vi "HFRR ADV v042.vi"() -> ()   [LabVIEW 2025] (continued)
        n1342 = case shown="True" w1655 {
          selector: w1655 -> [_ w1662]
          frame False {
          }
          frame True {
            n1343 = Not(x=w1662) -> (.not. x?=w1661:bool)
            n1344 = local write "LIVE FEED MIN TEMP"(w1661) -> ()
            n1345 = call "CAMERA LIVE FEED FGV.vi"("Enum - Menu"=CAMERA_LIVE_FEED_ENUM."CAMERA MINIMIZE") -> ()  [unwired: 9 in, 2 out]
          }
        }
        n1346 = case shown="True" w1653 {
          selector: w1653 -> [_ w1659]
          frame False {
          }
          frame True {
            n1347 = Not(x=w1659) -> (.not. x?=w1658:bool)
            n1348 = local write "CAMERA ROI MIN TEMP"(w1658) -> ()
            n1349 = call "IMAGE ANALYSIS.vi"("Enum"=POST_ANALYSIS_ENUM."MINIMIZE UI") -> ()  [unwired: 9 in, 2 out]
          }
        }
        n1350 = local write "CAMERA ROI MAX TEMP"(TRUE ("CAMERA ROI MAX TEMP")) -> ()
      }
      frame "Adv Scar" {
        n1351 = local read "CAMERA ROI MIN TEMP"() -> (w1663:bool)
        n1352 = case shown="True" "LIVE FEED MAX TEMP" {
          selector: "LIVE FEED MAX TEMP" -> [_ w1684]
          frame False {
          }
          frame True {
            n1353 = Not(x=w1684) -> (.not. x?=w1683:bool)
            n1354 = local write "LIVE FEED MAX TEMP"(w1683) -> ()
            n1355 = call "CAMERA LIVE FEED FGV.vi"("Enum - Menu"=CAMERA_LIVE_FEED_ENUM."CAMERA RESTORE") -> ("error out"=w1674:errorcluster)  [unwired: 9 in, 1 out]
            n1356 = Type Cast(type=30, x=0) -> (*(type *) &x=w1678:i32)
            n1357 = Add(x=w1678, y=48) -> (x+y=w1679:i32)
            n1358 = call "CAMERA LIVE FEED FGV.vi"("Enum - Menu"=CAMERA_LIVE_FEED_ENUM."CAMERA MODE SET", "error in (no error)"=w1674, "CAMERA MODE"=w1679) -> ("error out"=w1671:errorcluster)  [unwired: 7 in, 1 out]
            n1359 = call "CAMERA LIVE FEED FGV.vi"("Enum - Menu"=CAMERA_LIVE_FEED_ENUM."CAMERA GRAY", "error in (no error)"=w1671) -> ("error out"=w1670:errorcluster)  [unwired: 8 in, 1 out]
            n1360 = call "LIST FILE NAMES.vi"("error in (no error)"=w1670) -> ("error out"=w1680:errorcluster, "filenames"=w1681:string[])  [unwired: 9 in]
            n1361 = property on="FILE 3" class="CmbBox"(error in=w1680, "Strings[]"=w1681) -> ()  [unwired: 1 in, 2 out]
          }
        }
        n1362 = case shown="True" w1663 {
          selector: w1663 -> [_ w1669]
          frame False {
          }
          frame True {
            n1363 = Not(x=w1669) -> (.not. x?=w1668:bool)
            n1364 = local write "CAMERA ROI MIN TEMP"(w1668) -> ()
            n1365 = call "IMAGE ANALYSIS.vi"("Enum"=POST_ANALYSIS_ENUM."MINIMIZE UI") -> ()  [unwired: 9 in, 2 out]
          }
        }
        n1366 = local write "CAMERA ROI MAX TEMP"(TRUE ("CAMERA ROI MAX TEMP")) -> ()
        "LIVE FEED MIN TEMP" <- TRUE ("LIVE FEED MIN TEMP")
      }
      frame "Adv Scar Report" {
        n1367 = local read "CAMERA ROI MAX TEMP"() -> (w1685:bool)
        n1368 = local read "LIVE FEED MIN TEMP"() -> (w1687:bool)
        n1369 = local write "LIVE FEED MAX TEMP"(TRUE ("LIVE FEED MAX TEMP")) -> ()
        n1370 = case shown="True" w1687 {
          selector: w1687 -> [_ w1696]
          frame False {
          }
          frame True {
            n1371 = Not(x=w1696) -> (.not. x?=w1695:bool)
            n1372 = local write "LIVE FEED MIN TEMP"(w1695) -> ()
            n1373 = call "CAMERA LIVE FEED FGV.vi"("Enum - Menu"=CAMERA_LIVE_FEED_ENUM."CAMERA MINIMIZE") -> ()  [unwired: 9 in, 2 out]
          }
        }
        n1374 = case shown="True" w1685 {
          selector: w1685 -> [_ w1693]
          frame False {
          }
          frame True {
            n1375 = Not(x=w1693) -> (.not. x?=w1691:bool)
            n1376 = local write "CAMERA ROI MAX TEMP"(w1691) -> ()
            n1377 = call "IMAGE ANALYSIS.vi"("Enum"=POST_ANALYSIS_ENUM."SHOW UI") -> ("error out"=w1690:errorcluster)  [unwired: 9 in, 1 out]
            n1378 = call "LIST FILE NAMES.vi"("error in (no error)"=w1690) -> ("filenames"=w1689:string[])  [unwired: 9 in, 1 out]
            n1379 = property on="Test File List :" class="CmbBox"("Strings[]"=w1689) -> ()  [unwired: 2 in, 2 out]
          }
        }
        n1380 = local write "CAMERA ROI MIN TEMP"(TRUE ("CAMERA ROI MIN TEMP")) -> ()
      }
      frame "Compare Files" {
        n1381 = local read "LIVE FEED MIN TEMP"() -> (w1699:bool)
        n1382 = local write "LIVE FEED MAX TEMP"(TRUE ("LIVE FEED MAX TEMP")) -> ()
        n1383 = local read "CAMERA ROI MIN TEMP"() -> (w1697:bool)
        n1384 = case shown="True" w1699 {
          selector: w1699 -> [_ w1706]
          frame False {
          }
          frame True {
            n1385 = Not(x=w1706) -> (.not. x?=w1705:bool)
            n1386 = local write "LIVE FEED MIN TEMP"(w1705) -> ()
            n1387 = call "CAMERA LIVE FEED FGV.vi"("Enum - Menu"=CAMERA_LIVE_FEED_ENUM."CAMERA MINIMIZE") -> ()  [unwired: 9 in, 2 out]
          }
        }
        n1388 = case shown="True" w1697 {
          selector: w1697 -> [_ w1703]
          frame False {
          }
          frame True {
            n1389 = Not(x=w1703) -> (.not. x?=w1702:bool)
            n1390 = local write "CAMERA ROI MIN TEMP"(w1702) -> ()
            n1391 = call "IMAGE ANALYSIS.vi"("Enum"=POST_ANALYSIS_ENUM."MINIMIZE UI") -> ()  [unwired: 9 in, 2 out]
          }
        }
        n1392 = local write "CAMERA ROI MAX TEMP"(TRUE ("CAMERA ROI MAX TEMP")) -> ()
      }
      frame "About" {
        n1393 = local read "LIVE FEED MIN TEMP"() -> (w1709:bool)
        n1394 = local write "LIVE FEED MAX TEMP"(TRUE ("LIVE FEED MAX TEMP")) -> ()
        n1395 = local read "CAMERA ROI MIN TEMP"() -> (w1708:bool)
        n1396 = case shown="True" w1709 {
          selector: w1709 -> [_ w1716]
          frame False {
          }
          frame True {
            n1397 = Not(x=w1716) -> (.not. x?=w1715:bool)
            n1398 = local write "LIVE FEED MIN TEMP"(w1715) -> ()
            n1399 = call "CAMERA LIVE FEED FGV.vi"("Enum - Menu"=CAMERA_LIVE_FEED_ENUM."CAMERA MINIMIZE") -> ()  [unwired: 9 in, 2 out]
          }
        }
        n1400 = case shown="True" w1708 {
          selector: w1708 -> [_ w1713]
          frame False {
          }
          frame True {
            n1401 = Not(x=w1713) -> (.not. x?=w1712:bool)
            n1402 = local write "CAMERA ROI MIN TEMP"(w1712) -> ()
            n1403 = call "IMAGE ANALYSIS.vi"("Enum"=POST_ANALYSIS_ENUM."MINIMIZE UI") -> ()  [unwired: 9 in, 2 out]
          }
        }
        n1404 = local write "CAMERA ROI MAX TEMP"(TRUE ("CAMERA ROI MIN TEMP")) -> ()
      }
      frame "Advance" {
        n1405 = local read "LIVE FEED MIN TEMP"() -> (w1719:bool)
        n1406 = local write "LIVE FEED MAX TEMP"(TRUE ("LIVE FEED MAX TEMP")) -> ()
        n1407 = local read "CAMERA ROI MIN TEMP"() -> (w1717:bool)
        n1408 = case shown="True" w1719 {
          selector: w1719 -> [_ w1726]
          frame False {
          }
          frame True {
            n1409 = Not(x=w1726) -> (.not. x?=w1725:bool)
            n1410 = local write "LIVE FEED MIN TEMP"(w1725) -> ()
            n1411 = call "CAMERA LIVE FEED FGV.vi"("Enum - Menu"=CAMERA_LIVE_FEED_ENUM."CAMERA MINIMIZE") -> ()  [unwired: 9 in, 2 out]
          }
        }
        n1412 = local write "CAMERA ROI MAX TEMP"(TRUE ("CAMERA ROI MAX TEMP")) -> ()
        n1413 = case shown="True" w1717 {
          selector: w1717 -> [_ w1723]
          frame False {
          }
          frame True {
            n1414 = Not(x=w1723) -> (.not. x?=w1722:bool)
            n1415 = local write "CAMERA ROI MIN TEMP"(w1722) -> ()
            n1416 = call "IMAGE ANALYSIS.vi"("Enum"=POST_ANALYSIS_ENUM."MINIMIZE UI") -> ()  [unwired: 9 in, 2 out]
          }
        }
      }
      frame "Mooha" {
        n1417 = local read "LIVE FEED MIN TEMP"() -> (w1729:bool)
        n1418 = local write "LIVE FEED MAX TEMP"(TRUE ("LIVE FEED MAX TEMP")) -> ()
        n1419 = local read "CAMERA ROI MIN TEMP"() -> (w1727:bool)
        n1420 = case shown="True" w1729 {
          selector: w1729 -> [_ w1736]
          frame False {
          }
          frame True {
            n1421 = Not(x=w1736) -> (.not. x?=w1735:bool)
            n1422 = local write "LIVE FEED MIN TEMP"(w1735) -> ()
            n1423 = call "CAMERA LIVE FEED FGV.vi"("Enum - Menu"=CAMERA_LIVE_FEED_ENUM."CAMERA MINIMIZE") -> ()  [unwired: 9 in, 2 out]
          }
        }
        n1424 = local write "CAMERA ROI MAX TEMP"(TRUE ("CAMERA ROI MAX TEMP")) -> ()
        n1425 = case shown="True" w1727 {
          selector: w1727 -> [_ w1733]
          frame False {
          }
          frame True {
            n1426 = Not(x=w1733) -> (.not. x?=w1732:bool)
            n1427 = local write "CAMERA ROI MIN TEMP"(w1732) -> ()
            n1428 = call "IMAGE ANALYSIS.vi"("Enum"=POST_ANALYSIS_ENUM."MINIMIZE UI") -> ()  [unwired: 9 in, 2 out]
          }
        }
      }
    }
    n1429 = local read "Auto Start Test"() -> (w1474:bool)
    n1430 = case shown="True" "sign in temp" {
      frame False {
      }
      frame True {
        w1509 = 1 ("y")
        n1431 = local read "USERNAME"() -> (w1515:string)
        n1432 = local read "USER ID"() -> (w1512:string)
        n1433 = call <vilib>:"Trim Whitespace.vi"("string"=w1515) -> ("trimmed string"=w1514:string)  [unwired: 1 in]
        n1434 = call <vilib>:"Trim Whitespace.vi"("string"=w1512) -> ("trimmed string"=w1513:string)  [unwired: 1 in]
        n1435 = String Length(string=w1514) -> (length=w1511:i32)
        n1436 = String Length(string=w1513) -> (length=w1510:i32)
        n1437 = Greater?(x=w1511, y=w1509) -> (0:w1508:bool)
        n1438 = Greater?(x=w1510, y=w1509) -> (0:w1507:bool)
        n1439 = And(x=w1508, y=w1507) -> (x .and. y?=w1506:bool)
        n1440 = case shown="True" w1506 {
          frame False {
            n1441 = property on="Sign In" class="Bool (strict)"("DisabledEnum"=T19."Disabled" ("Disabled")) -> ()  [unwired: 2 in, 2 out]
          }
          frame True {
            n1442 = property on="Sign In" class="Bool (strict)"("DisabledEnum"=T19."Enabled" ("Disabled")) -> ()  [unwired: 2 in, 2 out]
          }
        }
      }
    }
    n1443 = local read "Air Temperature"() -> (w1491:bool)
    n1444 = local read "Coefficient Of Friction"() -> (w1492:bool)
    n1445 = case shown="False" w1474 {
      frame False {
        n1446 = local read "Auto stop temp"() -> (w1503:bool)
        n1447 = case shown="True" w1503 {
          frame False {
          }
          frame True {
            n1448 = local write "Auto Start Temp"(FALSE ("Auto Start Temp")) -> ()
          }
        }
      }
      frame True {
        "Auto stop temp" <- TRUE ("Auto stop temp")
      }
    }
    n1449 = local read "Humidity 3"() -> (w1490:bool)
    n1450 = case shown="\"HOME\"" w1500 {
      frame "HOME" {
        n1451 = local write "main tab sub"(enum32{"Page 1", "Page 2"}."Page 1" ("main tab sub")) -> ()
      }
      frame Default {
        n1452 = local write "main tab sub"(enum32{"Page 1", "Page 2"}."Page 2" ("main tab sub")) -> ()
      }
    }
    n1453 = case shown="True" w1499 {
      selector: w1499 -> [_ w1851]
      frame False {
      }
      frame True {
        n1454 = Not(x=w1851) -> (.not. x?=w1850:bool)
        n1455 = local write "Sign In"(w1850) -> ()
        n1456 = local write "Main Dashboard Buttons"(T25."Test Setup" ("Main Dashboard Buttons")) -> ()
      }
    }
    n1457 = case shown="\"Numeric Display\", Default" "Num/Graph" {
      frame "Numeric Display", Default {
        n1458 = property on="Single/Multiple" class="RadioBtnsControl (strict)"("Visible"=FALSE) -> ()  [unwired: 2 in, 2 out]
        n1459 = property on="Single - Graph" class="Ring (strict)"("Visible"=FALSE) -> ()  [unwired: 2 in, 2 out]
        n1460 = local write "Main Tab Display"(T4."Dashboard 1" ("Main Tab Display")) -> ()
      }
      frame "Graph Display" {
        n1461 = property on="Single/Multiple" class="RadioBtnsControl (strict)"("Visible"=TRUE) -> ()  [unwired: 2 in, 2 out]
        n1462 = case shown="\"Multiple\"" "Single/Multiple" {
          frame "Single ", Default {
            n1463 = property on="Single - Graph" class="Ring (strict)"("Visible"=TRUE) -> ()  [unwired: 2 in, 2 out]
            n1464 = local write "Main Tab Display"(T4."Dashboard 3" ("Main Tab Display")) -> ()
          }
          frame "Multiple" {
            n1465 = property on="Single - Graph" class="Ring (strict)"("Visible"=FALSE) -> ()  [unwired: 2 in, 2 out]
            n1466 = local write "Main Tab Display"(T4."Dashboard 2" ("Main Tab Display")) -> ()
          }
        }
      }
    }
    n1467 = local read "Stroke"() -> (w1489:bool)
    n1468 = local read "USERNAME"() -> (w1494:string)
    n1469 = case shown="True" w1492 {
      selector: w1492 -> [_ w1776]
      frame False {
      }
      frame True {
        n1470 = Not(x=w1776) -> (.not. x?=w1775:bool)
        n1471 = local write "Coefficient Of Friction"(w1775) -> ()
        n1472 = local write "Tab Control 2"(T6."Coefficient Of Friction" ("Tab Control 2")) -> ()
      }
    }
    n1473 = case shown="True" w1491 {
      selector: w1491 -> [_ w1773]
      frame False {
      }
      frame True {
        n1474 = Not(x=w1773) -> (.not. x?=w1771:bool)
        n1475 = local write "Air Temperature"(w1771) -> ()
        n1476 = local write "Tab Control 2"(T6."Air Temperature" ("Tab Control 2")) -> ()
      }
    }
    n1477 = case shown="True" w1489 {
      selector: w1489 -> [_ w1767]
      frame False {
      }
      frame True {
        n1478 = Not(x=w1767) -> (.not. x?=w1765:bool)
        n1479 = local write "Stroke"(w1765) -> ()
        n1480 = local write "Tab Control 2"(T6."Stroke" ("Tab Control 2")) -> ()
      }
    }
    n1481 = local write "tested by"(w1494) -> ()
    n1482 = case shown="True" w1490 {
      selector: w1490 -> [_ w1770]
      frame False {
      }
      frame True {
        n1483 = Not(x=w1770) -> (.not. x?=w1768:bool)
        n1484 = local write "Humidity 3"(w1768) -> ()
        n1485 = local write "Tab Control 2"(T6."Humidity" ("Tab Control 2")) -> ()
      }
    }
    n1486 = case shown="\"Calibration\"" "Main Dashboard Buttons" {
      tunnel: [T2."HOME" ("Main Tab") T2."Test Setup" ("Main Tab") T2."Acquire" ("Main Tab") T2."Adv Scar" ("Main Tab") T2."Adv Scar Report" ("Main Tab") T2."Compare Files" ("Main Tab") T2."Calibration" ("Main Tab") T2."About" ("Main Tab") T2."Advance" ("Main Tab")] -> w1473
      frame "Home", Default {
      }
      frame "Test Setup" {
      }
      frame "Dashboard" {
      }
      frame "Imaging" {
      }
      frame "Report" {
      }
      frame "Analysis" {
      }
      frame "Calibration" {
      }
      frame "About" {
      }
      frame "Advance" {
      }
    }
    n1487 = Wait (ms)(milliseconds to wait=u32 100) -> ()  [unwired: 1 out]
    n1488 = local read "Main Tab Display"() -> (w1493:T4)
    n1489 = local write "Main Tab"(w1473) -> ()
    n1490 = case shown="\"Dashboard 3\"" w1493 {
      frame "Dashboard 1", Default {
        n1491 = property on="Reset Graph" class="Bool (strict)"("Visible"=FALSE) -> ()  [unwired: 2 in, 2 out]
      }
      frame "Dashboard 2" {
        n1492 = property on="Reset Graph" class="Bool (strict)"("Visible"=TRUE) -> ()  [unwired: 2 in, 2 out]
      }
      frame "Dashboard 3" {
        n1493 = property on="Reset Graph" class="Bool (strict)"("Visible"=TRUE) -> ()  [unwired: 2 in, 2 out]
      }
    }
    n1494 = local read "SCAR MEASURMENT"() -> (w1481:enum32{"Auto Scar", "Manual Scar"})
    n1495 = local read "Humidity"() -> (w1495:bool)
    n1496 = local read "Cap Live Image"() -> (w1478:bool)
    n1497 = local read "Sample Temperature"() -> (w1488:bool)
    n1498 = local read "Air Temp vs Humidity"() -> (w1486:bool)
    n1499 = local read "Frequency"() -> (w1487:bool)
    n1500 = case shown="False" w1495 {
      frame False {
        n1501 = local write "Humidity On Command"(TRUE ("Humidity On Command")) -> ()
        n1502 = case shown="True" "Humidity Off Command" {
          selector: "Humidity Off Command" -> [_ w1783]
          frame False {
          }
          frame True {
            n1503 = stacked-sequence {
              frame #0 {
                n1504 = local read "WriteHumidity"() -> (w1785:string[])
                n1505 = Insert Into Array(array=w1785, new element="R;1" ("new element/subarray")) -> (w1784:string[])  [unwired: 1 in]
                n1506 = local write "WriteHumidity"(w1784) -> ()
              }
              frame #1 {
                n1507 = Wait (ms)(milliseconds to wait=u32 500) -> ()  [unwired: 1 out]
              }
              frame #2 {
                n1508 = local read "WriteHumidity"() -> (w1789:string[])
                n1509 = local read "EVENT LOG"() -> (w1793:string)
                n1510 = call "Event Log.vi"("Content"="Humidity Control Off" ("string"), "EVENT LOG"=w1793) -> ("EVENT LOG"=w1794:string)  [unwired: 8 in, 1 out]
                n1511 = local write "EVENT LOG"(w1794) -> ()
                n1512 = Insert Into Array(array=w1789, new element="R;1" ("new element/subarray")) -> (w1790:string[])  [unwired: 1 in]
                n1513 = local write "WriteHumidity"(w1790) -> ()
                n1514 = local write "Humidity 2"(TRUE ("Humidity")) -> ()
              }
            }
            n1515 = Not(x=w1783) -> (.not. x?=w1782:bool)
            n1516 = local write "Humidity Off Command"(w1782) -> ()
          }
        }
      }
      frame True {
        n1517 = local write "Humidity Off Command"(TRUE ("Humidity Off Command")) -> ()
        n1518 = case shown="False" "Humidity On Command" {
          selector: "Humidity On Command" -> [_ w1798]
          frame False {
          }
          frame True {
            n1519 = stacked-sequence {
              frame #0 {
                n1520 = local read "Set Rh"() -> (w1804:dbl)
                n1521 = local read "WriteHumidity"() -> (w1800:string[])
                n1522 = Number To Fractional String(number=w1804, precision (6)=i16 2) -> (F-format string=w1805:string)  [unwired: 2 in]
                n1523 = Concatenate Strings("M;" ("new element/subarray"), w1805) -> (w1803:string)
                n1524 = Insert Into Array(array=w1800, new element=w1803) -> (w1799:string[])  [unwired: 1 in]
                n1525 = local write "WriteHumidity"(w1799) -> ()
              }
              frame #1 {
                n1526 = Wait (ms)(milliseconds to wait=u32 500) -> ()  [unwired: 1 out]
              }
              frame #2 {
                n1527 = local read "WriteHumidity"() -> (w1808:string[])
                n1528 = local read "Set Rh"() -> (w1812:dbl)
                n1529 = Number To Fractional String(number=w1812, precision (6)=i16 2) -> (F-format string=w1813:string)  [unwired: 2 in]
                n1530 = Concatenate Strings("M;" ("new element/subarray"), w1813) -> (w1811:string)
                n1531 = Insert Into Array(array=w1808, new element=w1811) -> (w1807:string[])  [unwired: 1 in]
                n1532 = local write "WriteHumidity"(w1807) -> ()
              }
              frame #3 {
                n1533 = Wait (ms)(milliseconds to wait=u32 500) -> ()  [unwired: 1 out]
              }
              frame #4 {
                (unwired) "% RH" ("string")
                (unwired) i16 2 ("precision (6)")
                (unwired) "M;" ("new element/subarray")
                n1534 = local read "Set Rh"() -> (w1822:dbl)
                n1535 = local read "WriteHumidity"() -> (w1815:string[])
                n1536 = Number To Fractional String(number=w1822, precision (6)=i16 2) -> (F-format string=w1819:string)  [unwired: 2 in]
                n1537 = Concatenate Strings("M;" ("new element/subarray"), w1819) -> (w1823:string)
                n1538 = Concatenate Strings("Humidity Set to : " ("string"), w1819, "% RH" ("string")) -> (w1817:string)
                n1539 = Insert Into Array(array=w1815, new element=w1823) -> (w1816:string[])  [unwired: 1 in]
                n1540 = disable-structure shown="Enabled" {
                  frame Enabled {
                    n1541 = local read "EVENT LOG"() -> (w1826:string)
                    n1542 = call "Event Log.vi"("Content"="Humidity Control On", "EVENT LOG"=w1826) -> ("EVENT LOG"=w1827:string)  [unwired: 8 in, 1 out]
                    n1543 = local write "EVENT LOG"(w1827) -> ()
                  }
                  frame Disabled {
                  }
                }
                n1544 = disable-structure shown="Enabled" {
                  disable-tunnel: w1817 -> [_ _]
                  frame Enabled {
                    n1545 = local read "EVENT LOG"() -> (w1829:string)
                    n1546 = call "Event Log.vi"("Content"="Humidity Control On", "EVENT LOG"=w1829) -> ("EVENT LOG"=w1830:string)  [unwired: 8 in, 1 out]
                    n1547 = local write "EVENT LOG"(w1830) -> ()
                  }
                  frame Disabled {
                  }
                }
                n1548 = local write "WriteHumidity"(w1816) -> ()
              }
            }
            n1549 = Not(x=w1798) -> (.not. x?=w1797:bool)
            n1550 = local write "Humidity On Command"(w1797) -> ()
          }
        }
      }
    }
    n1551 = Equal?(x=w1481, y=enum32{"Auto Scar", "Manual Scar"}."Auto Scar" ("SCAR MEASURMENT")) -> (x = y?=w1477:bool)
    n1552 = local read "TEST STANDARD"() -> (w1484:T3)
    n1553 = And(x=w1478, y=w1477) -> (x .and. y?=w1479:bool)
    n1554 = case shown="True" w1479 {
      selector: w1479 -> [_ w1582]
      tunnel: errorcluster {"status"=FALSE, "code"=0, "source"=""} ("error in (no error) 3") -> [_ w1583]
      frame False {
      }
      frame True {
        n1555 = stacked-sequence {
          tunnel: w1583 -> [_ _ _ _ _ _ _ w1631]
          tunnel: w1582 -> [_ _ _ _ _ w1612 _ _]
          frame #0 {
            n1556 = call "CAMERA LIVE FEED FGV.vi"("Enum - Menu"=CAMERA_LIVE_FEED_ENUM."CAMERA MINIMIZE") -> ()  [unwired: 9 in, 2 out]
          }
          frame #1 {
            n1557 = property on="Auto Scar Check  2" class="Clust (strict)"("Visible"=TRUE) -> ()  [unwired: 2 in, 2 out]
          }
          frame #2 {
            n1558 = String To Path(string="C:\\LAB-IQ\\Image Calibrate v01.dcf") -> (path=w1588:path)
            n1559 = Open/Create/Replace File ("Open File")(file path (use dialog)=w1588) -> (refnum out=w1589:refnum<file>)  [unwired: 5 in, 2 out]
            n1560 = for {
              N: 4 -> [_]
              tunnel: w1589 -> [w1595]
              i -> [w1591]
              n1561 = Read from Text File ("Read File")(file (use dialog)=w1595) -> (text=w1596:string)  [unwired: 3 in, 3 out]
              n1562 = String Subset(string=w1596, offset (0)=6, length (rest)=10 ("length (rest)")) -> (substring=w1592:string)
              n1563 = Fract/Exp String To Number(string=w1592) -> (number=w1590:dbl)  [unwired: 3 in, 1 out]
              n1564 = case shown="0" w1591 {
                tunnel: w1590 -> [w1597 w1598 _ w1599 _]
                frame 0 {
                  "5x Gain" <- w1597
                }
                frame 1 {
                  "10x Gain" <- w1598
                }
                frame 2 {
                }
                frame 3 {
                  "100x gain" <- w1599
                }
                frame 4, Default {
                }
              }
            }
          }
          frame #3 {
            n1565 = local read "FILE 3"() -> (w1605:string)
            n1566 = call <vilib>:"Trim Whitespace.vi"("string"="C:\\LAB-IQ\\images\\") -> ("trimmed string"=w1607:string)  [unwired: 1 in]
            n1567 = String To Path(string=w1607) -> (path=w1606:path)
            n1568 = Concatenate Strings(w1605, ".png" ("string")) -> (w1604:string)
            n1569 = Build Path(base path=w1606, name or relative path=w1604) -> (appended path=w1602:path)
            "Image path" <- w1602
            n1570 = Path To String(path=w1602) -> (string=w1601:string)
            n1571 = call "CAMERA LIVE FEED FGV.vi"("Enum - Menu"=CAMERA_LIVE_FEED_ENUM."CAMERA SAVE", "Image Path"=w1601) -> ()  [unwired: 8 in, 2 out]
          }
          frame #4 {
            n1572 = One Button Dialog(message="Image saved successfully") -> ()  [unwired: 1 in, 1 out]
          }
          frame #5 {
            n1573 = local read "TEST STANDARD"() -> (w1611:T3)
            n1574 = local read "Magnification len live scar"() -> (w1623:string)
            n1575 = Not(x=w1612) -> (.not. x?=w1613:bool)
            n1576 = local write "Cap Live Image"(w1613) -> ()
            n1577 = case shown="\"ISO 12156\"" w1611 {
              tunnel: ["ASTM D6079" "ISO 12156"] -> w1610
              frame "ASTM D6079", Default {
              }
              frame "ISO 12156" {
              }
            }
            n1578 = case shown="\"5x\", Default" w1623 {
              tunnel: [w1626 w1627] -> w1622
              frame "5x", Default {
                n1579 = local read "5x Gain"() -> (w1626:dbl)
              }
              frame "10x" {
                # "5x"
                n1580 = local read "10x Gain"() -> (w1627:dbl)
              }
            }
            n1581 = local read "Image path"() -> (w1621:path)
            n1582 = local read "FILE 3"() -> (w1614:string)
            n1583 = call "EDGE DETCTION.vi"("GAIN VALUE"=w1622, "Image Path"=w1621) -> ("error out"=w1620:errorcluster, "return value"=w1619:cluster{string, string, dbl, dbl, dbl})  [unwired: 8 in]
            n1584 = Bundle By Name(cluster=T26 {"File Name"="", "Test Method"="", "Operator"="", "Fuel Description"="", "Date and time"=""} ("Main Ref"), "File Name"=w1614, "Test Method"=w1610) -> (w1615:T26)
            n1585 = call "duf file read.vi"("error in (no error)"=w1620, "Main Ref"=w1615) -> ("error out"=w1618:errorcluster, "Main Ref 2"=w1616:T26)  [unwired: 8 in]
            n1586 = call "EDGE DETECTION REPORT.vi"("error in (no error)"=w1618, "return value 2"=w1619, "Main Ref"=w1616) -> ()  [unwired: 8 in, 1 out]
          }
          frame #6 {
            n1587 = property on="Auto Scar Check  2" class="Clust (strict)"("Visible"=FALSE) -> ()  [unwired: 2 in, 2 out]
          }
          frame #7 {
            n1588 = call "CAMERA LIVE FEED FGV.vi"("Enum - Menu"=CAMERA_LIVE_FEED_ENUM."CAMERA MINIMIZE", "error in (no error)"=w1631) -> ()  [unwired: 8 in, 2 out]
            n1589 = local write "Main Dashboard Buttons"(T1."Home" ("Main Dashboard Buttons")) -> ()
            n1590 = local write "Main Tab"(T2."HOME" ("Main Tab")) -> ()
          }
        }
      }
    }
    n1591 = local read "Heater Button"() -> (w1485:bool)
    n1592 = case shown="True" w1487 {
      selector: w1487 -> [_ w1761]
      frame False {
      }
      frame True {
        n1593 = Not(x=w1761) -> (.not. x?=w1759:bool)
        n1594 = local write "Frequency"(w1759) -> ()
        n1595 = local write "Tab Control 2"(T6."Frequency" ("Tab Control 2")) -> ()
      }
    }
    n1596 = case shown="True" w1486 {
      selector: w1486 -> [_ w1758]
      frame False {
      }
      frame True {
        n1597 = Not(x=w1758) -> (.not. x?=w1756:bool)
        n1598 = local write "Air Temp vs Humidity"(w1756) -> ()
        n1599 = local write "Tab Control 2"(T6."Air Temp vs Rh" ("Tab Control 2")) -> ()
      }
    }
    n1600 = case shown="True" w1488 {
      selector: w1488 -> [_ w1764]
      frame False {
      }
      frame True {
        n1601 = Not(x=w1764) -> (.not. x?=w1762:bool)
        n1602 = local write "Sample Temperature"(w1762) -> ()
        n1603 = local write "Tab Control 2"(T6."Sample Temperature" ("Tab Control 2")) -> ()
      }
    }
    n1604 = case shown="\"Custom\"" w1484 {
      frame "ASTM D6079", Default {
        w1737 = "ASTM D6079 TEST CONDITIONS" ("Standard 2")
        n1605 = local write "Standard 2"(w1737) -> ()
        n1606 = local write "Standard"(w1737) -> ()
      }
      frame "ISO 12156" {
        w1738 = "ISO 12156 TEST CONDITIONS" ("Standard 2")
        n1607 = local write "Standard 2"(w1738) -> ()
        n1608 = local write "Standard"(w1738) -> ()
      }
      frame "CEC F-096-A-06" {
        w1739 = "CEC F-096-A-06 TEST CONDITIONS" ("Standard 2")
        n1609 = local write "Standard 2"(w1739) -> ()
        n1610 = local write "Standard"(w1739) -> ()
      }
      frame "Custom" {
        w1740 = "CUSTOM TEST CONDITIONS" ("Standard 2")
        n1611 = local write "Standard 2"(w1740) -> ()
        n1612 = local write "Standard"(w1740) -> ()
      }
    }
    n1613 = case shown="True" w1485 {
      frame False {
        n1614 = local write "Temperature On Command"(TRUE ("Temperature On Command")) -> ()
        n1615 = case shown="True" "Temperature Off Command" {
          selector: "Temperature Off Command" -> [_ w1744]
          frame False {
          }
          frame True {
            n1616 = Not(x=w1744) -> (.not. x?=w1743:bool)
            n1617 = local read "EVENT LOG"() -> (w1747:string)
            n1618 = local write "Temperature Off Command"(w1743) -> ()
            n1619 = call "Event Log.vi"("Content"="Heater Off", "EVENT LOG"=w1747) -> ("EVENT LOG"=w1746:string)  [unwired: 8 in, 1 out]
            n1620 = local write "EVENT LOG"(w1746) -> ()
          }
        }
      }
      frame True {
        n1621 = local write "Temperature Off Command"(TRUE ("Temperature Off Command")) -> ()
        n1622 = case shown="True" "Temperature On Command" {
          selector: "Temperature On Command" -> [_ w1751]
          frame False {
          }
          frame True {
            n1623 = Not(x=w1751) -> (.not. x?=w1750:bool)
            n1624 = local write "Temperature On Command"(w1750) -> ()
            n1625 = disable-structure shown="Enabled" {
              disable-tunnel: "Heater On" -> [w1753 _]
              frame Enabled {
                n1626 = local read "EVENT LOG"() -> (w1754:string)
                n1627 = call "Event Log.vi"("Content"=w1753, "EVENT LOG"=w1754) -> ("EVENT LOG"=w1755:string)  [unwired: 8 in, 1 out]
                n1628 = local write "EVENT LOG"(w1755) -> ()
              }
              frame Disabled {
              }
            }
          }
        }
      }
    }
    n1629 = local read "Main Tab"() -> (w1476:T2)
    n1630 = case shown="\"About\"" w1476 {
      frame "HOME", Default {
        w1518 = T19."Enabled" ("Disabled")
        n1631 = local read "Service Password enable"() -> (w1520:bool)
        n1632 = property on="Imaging" class="Bool (strict)"("DisabledEnum"=w1518) -> ()  [unwired: 2 in, 2 out]
        n1633 = property on="Dashboard" class="Bool (strict)"("DisabledEnum"=w1518) -> ()  [unwired: 2 in, 2 out]
        n1634 = property on="Test Setup" class="Bool (strict)"("DisabledEnum"=w1518) -> ()  [unwired: 2 in, 2 out]
        n1635 = property on="Analysis" class="Bool (strict)"("DisabledEnum"=w1518) -> ()  [unwired: 2 in, 2 out]
        n1636 = property on="Home" class="Bool (strict)"("DisabledEnum"=w1518) -> ()  [unwired: 2 in, 2 out]
        n1637 = property on="Report" class="Bool (strict)"("DisabledEnum"=w1518) -> ()  [unwired: 2 in, 2 out]
        n1638 = property on="Main Dashboard Buttons" class="RadioBtnsControl (strict)"("DisabledEnum"=w1518) -> ()  [unwired: 2 in, 2 out]
        n1639 = property on="Calibration" class="Bool (strict)"("DisabledEnum"=w1518) -> ()  [unwired: 2 in, 2 out]
        n1640 = case shown="True" w1520 {
          tunnel: [T19."Disabled" ("Disabled") T19."Enabled" ("Disabled")] -> w1519
          frame False {
          }
          frame True {
          }
        }
        n1641 = property on="About" class="Bool (strict)"("DisabledEnum"=w1519) -> ()  [unwired: 2 in, 2 out]
      }
      frame "Test Setup" {
        w1525 = T19."Enabled" ("Disabled")
        n1642 = local read "Service Password enable"() -> (w1524:bool)
        n1643 = property on="Dashboard" class="Bool (strict)"("DisabledEnum"=T19."Disabled" ("Disabled")) -> ()  [unwired: 2 in, 2 out]
        n1644 = property on="Imaging" class="Bool (strict)"("DisabledEnum"=w1525) -> ()  [unwired: 2 in, 2 out]
        n1645 = property on="Analysis" class="Bool (strict)"("DisabledEnum"=w1525) -> ()  [unwired: 2 in, 2 out]
        n1646 = property on="Home" class="Bool (strict)"("DisabledEnum"=w1525) -> ()  [unwired: 2 in, 2 out]
        n1647 = property on="Report" class="Bool (strict)"("DisabledEnum"=w1525) -> ()  [unwired: 2 in, 2 out]
        n1648 = property on="Test Setup" class="Bool (strict)"("DisabledEnum"=w1525) -> ()  [unwired: 2 in, 2 out]
        n1649 = case shown="True" w1524 {
          tunnel: [T19."Disabled" ("Disabled") T19."Enabled" ("Disabled")] -> w1523
          frame False {
          }
          frame True {
          }
        }
        n1650 = property on="About" class="Bool (strict)"("DisabledEnum"=w1523) -> ()  [unwired: 2 in, 2 out]
      }
      frame "Adv Scar" {
        w1532 = T19."Enabled" ("Disabled")
        n1651 = property on="Dashboard" class="Bool (strict)"("DisabledEnum"=T19."Disabled" ("Disabled")) -> ()  [unwired: 2 in, 2 out]
        n1652 = property on="Imaging" class="Bool (strict)"("DisabledEnum"=w1532) -> ()  [unwired: 2 in, 2 out]
        n1653 = property on="Analysis" class="Bool (strict)"("DisabledEnum"=w1532) -> ()  [unwired: 2 in, 2 out]
        n1654 = property on="Home" class="Bool (strict)"("DisabledEnum"=w1532) -> ()  [unwired: 2 in, 2 out]
        n1655 = property on="Report" class="Bool (strict)"("DisabledEnum"=w1532) -> ()  [unwired: 2 in, 2 out]
        n1656 = property on="Test Setup" class="Bool (strict)"("DisabledEnum"=w1532) -> ()  [unwired: 2 in, 2 out]
        n1657 = local read "Service Password enable"() -> (w1530:bool)
        n1658 = case shown="True" w1530 {
          tunnel: [T19."Disabled" ("Disabled") T19."Enabled" ("Disabled")] -> w1529
          frame False {
          }
          frame True {
          }
        }
        n1659 = property on="About" class="Bool (strict)"("DisabledEnum"=w1529) -> ()  [unwired: 2 in, 2 out]
      }
      frame "Calibration" {
        w1535 = T19."Enabled" ("Disabled")
        n1660 = property on="Dashboard" class="Bool (strict)"("DisabledEnum"=T19."Disabled" ("Disabled")) -> ()  [unwired: 2 in, 2 out]
        n1661 = property on="Imaging" class="Bool (strict)"("DisabledEnum"=w1535) -> ()  [unwired: 2 in, 2 out]
        n1662 = property on="Analysis" class="Bool (strict)"("DisabledEnum"=w1535) -> ()  [unwired: 2 in, 2 out]
        n1663 = property on="Home" class="Bool (strict)"("DisabledEnum"=w1535) -> ()  [unwired: 2 in, 2 out]
        n1664 = property on="Report" class="Bool (strict)"("DisabledEnum"=w1535) -> ()  [unwired: 2 in, 2 out]
        n1665 = property on="Test Setup" class="Bool (strict)"("DisabledEnum"=w1535) -> ()  [unwired: 2 in, 2 out]
        n1666 = local read "Service Password enable"() -> (w1537:bool)
        n1667 = property on="Calibration" class="Bool (strict)"("DisabledEnum"=w1535) -> ()  [unwired: 2 in, 2 out]
        n1668 = case shown="True" w1537 {
          tunnel: [T19."Disabled" ("Disabled") T19."Enabled" ("Disabled")] -> w1536
          frame False {
          }
          frame True {
          }
        }
        n1669 = property on="About" class="Bool (strict)"("DisabledEnum"=w1536) -> ()  [unwired: 2 in, 2 out]
      }
      frame "Adv Scar Report" {
        w1543 = T19."Enabled" ("Disabled")
        n1670 = property on="Dashboard" class="Bool (strict)"("DisabledEnum"=T19."Disabled" ("Disabled")) -> ()  [unwired: 2 in, 2 out]
        n1671 = property on="Imaging" class="Bool (strict)"("DisabledEnum"=w1543) -> ()  [unwired: 2 in, 2 out]
        n1672 = property on="Analysis" class="Bool (strict)"("DisabledEnum"=w1543) -> ()  [unwired: 2 in, 2 out]
        n1673 = property on="Home" class="Bool (strict)"("DisabledEnum"=w1543) -> ()  [unwired: 2 in, 2 out]
        n1674 = property on="Report" class="Bool (strict)"("DisabledEnum"=w1543) -> ()  [unwired: 2 in, 2 out]
        n1675 = property on="Test Setup" class="Bool (strict)"("DisabledEnum"=w1543) -> ()  [unwired: 2 in, 2 out]
        n1676 = local read "Service Password enable"() -> (w1542:bool)
        n1677 = case shown="True" w1542 {
          tunnel: [T19."Disabled" ("Disabled") T19."Enabled" ("Disabled")] -> w1541
          frame False {
          }
          frame True {
          }
        }
        n1678 = property on="About" class="Bool (strict)"("DisabledEnum"=w1541) -> ()  [unwired: 2 in, 2 out]
      }
      frame "Compare Files" {
        w1549 = T19."Enabled" ("Disabled")
        n1679 = local read "Service Password enable"() -> (w1548:bool)
        n1680 = property on="Dashboard" class="Bool (strict)"("DisabledEnum"=T19."Disabled" ("Disabled")) -> ()  [unwired: 2 in, 2 out]
        n1681 = property on="Imaging" class="Bool (strict)"("DisabledEnum"=w1549) -> ()  [unwired: 2 in, 2 out]
        n1682 = property on="Analysis" class="Bool (strict)"("DisabledEnum"=w1549) -> ()  [unwired: 2 in, 2 out]
        n1683 = property on="Home" class="Bool (strict)"("DisabledEnum"=w1549) -> ()  [unwired: 2 in, 2 out]
        n1684 = property on="Report" class="Bool (strict)"("DisabledEnum"=w1549) -> ()  [unwired: 2 in, 2 out]
        n1685 = property on="Test Setup" class="Bool (strict)"("DisabledEnum"=w1549) -> ()  [unwired: 2 in, 2 out]
        n1686 = case shown="True" w1548 {
          tunnel: [T19."Disabled" ("Disabled") T19."Enabled" ("Disabled")] -> w1547
          frame False {
          }
          frame True {
          }
        }
        n1687 = property on="About" class="Bool (strict)"("DisabledEnum"=w1547) -> ()  [unwired: 2 in, 2 out]
      }
      frame "Acquire" {
        n1688 = local read "Service Password enable"() -> (w1554:bool)
        n1689 = property on="Test Setup" class="Bool (strict)"("DisabledEnum"=T19."Disabled" ("Disabled")) -> ()  [unwired: 2 in, 2 out]
        n1690 = local read "Auto Start Test"() -> (w1556:bool)
        n1691 = local read "RUN"() -> (w1558:bool)
        n1692 = case shown="True" w1554 {
          tunnel: [T19."Disabled" ("Disabled") T19."Enabled" ("Disabled")] -> w1555
          frame False {
          }
          frame True {
          }
        }
        n1693 = Or(x=w1558, y=w1556) -> (x .or. y?=w1557:bool)
        n1694 = case shown="True" w1557 {
          tunnel: [T19."Enabled" ("Disabled") T19."Disabled" ("Disabled")] -> w1553
          frame False {
          }
          frame True {
          }
        }
        n1695 = property on="About" class="Bool (strict)"("DisabledEnum"=w1555) -> ()  [unwired: 2 in, 2 out]
        n1696 = property on="Imaging" class="Bool (strict)"("DisabledEnum"=w1553) -> ()  [unwired: 2 in, 2 out]
        n1697 = property on="Dashboard" class="Bool (strict)"("DisabledEnum"=w1553) -> ()  [unwired: 2 in, 2 out]
        n1698 = property on="Analysis" class="Bool (strict)"("DisabledEnum"=w1553) -> ()  [unwired: 2 in, 2 out]
        n1699 = property on="Home" class="Bool (strict)"("DisabledEnum"=w1553) -> ()  [unwired: 2 in, 2 out]
        n1700 = property on="Report" class="Bool (strict)"("DisabledEnum"=w1553) -> ()  [unwired: 2 in, 2 out]
        n1701 = property on="Calibration" class="Bool (strict)"("DisabledEnum"=w1553) -> ()  [unwired: 2 in, 2 out]
      }
      frame "About" {
        n1702 = local read "FILE"() -> (w1572:string)
        n1703 = local read "TEST FILE NAM,E SAVED"() -> (w1565:bool)
        n1704 = call <vilib>:"Trim Whitespace.vi"("string"=w1572) -> ("trimmed string"=w1571:string)  [unwired: 1 in]
        n1705 = local read "Auto Start Test"() -> (w1575:bool)
        n1706 = String Length(string=w1571) -> (length=w1570:i32)
        n1707 = Greater?(x=w1570, y=1) -> (0:w1567:bool)
        n1708 = And(x=w1567, y=w1565) -> (x .and. y?=w1566:bool)
        n1709 = local read "RUN"() -> (w1577:bool)
        n1710 = case shown="True" w1566 {
          tunnel: [T19."Disabled" ("Disabled") T19."Enabled" ("Disabled")] -> w1568
          frame False {
          }
          frame True {
          }
        }
        n1711 = Or(x=w1577, y=w1575) -> (x .or. y?=w1576:bool)
        n1712 = property on="About" class="Bool (strict)"("DisabledEnum"=T19."Enabled" ("Disabled")) -> ()  [unwired: 2 in, 2 out]
        n1713 = case shown="False" w1576 {
          tunnel: [T19."Enabled" ("Disabled") T19."Disabled" ("Disabled")] -> w1574
          frame False {
          }
          frame True {
          }
        }
        n1714 = property on="Dashboard" class="Bool (strict)"("DisabledEnum"=w1568) -> ()  [unwired: 2 in, 2 out]
        n1715 = property on="Test Setup" class="Bool (strict)"("DisabledEnum"=T19."Disabled" ("Disabled")) -> ()  [unwired: 2 in, 2 out]
        n1716 = property on="Imaging" class="Bool (strict)"("DisabledEnum"=w1574) -> ()  [unwired: 2 in, 2 out]
        n1717 = property on="Analysis" class="Bool (strict)"("DisabledEnum"=w1574) -> ()  [unwired: 2 in, 2 out]
        n1718 = property on="Home" class="Bool (strict)"("DisabledEnum"=w1574) -> ()  [unwired: 2 in, 2 out]
        n1719 = property on="Report" class="Bool (strict)"("DisabledEnum"=w1574) -> ()  [unwired: 2 in, 2 out]
      }
    }
    n1720 = local read "Quit"() -> (w1502:bool)
    "Single" <- "Single - Graph"
  }
  n1721 = disable-structure shown="Disabled" {
    disable-tunnel: [w1855 _] -> w44
    disable-tunnel: _ -> [w1854 _]
    frame Disabled {
      n1722 = while {
        tunnel: w1854 -> [_]
        tunnel: [w1856] -> w1855
        tunnel: [w1857] -> _
        i -> [w1857]
        stop <- w1856 stop-if-true
        w1873 = u16 10 items=["1.0"=10, "1.5"=15, "2.0"=20] ("stop bits (10: 1 bit)")
        n1723 = Wait (ms)(milliseconds to wait=u32 10) -> ()  [unwired: 1 out]
        n1724 = call-poly "VISA Configure Serial Port"("VISA resource name"=refnum<visa-resource-name> "ASRL1::INSTR" ("COM PORT"), "timeout (10sec)"=u32 10, "baud rate (9600)"=u32 57600, "data bits (8)"=u16 8, "stop bits (10: 1 bit)"=w1873) -> ("VISA resource name out"=w1859:refnum<visa-resource-name>, "error out"=w1868:errorcluster)  [unwired: 9 in]
        n1725 = VISA Read(VISA resource name=w1859, byte count=u32 2 ("byte count (0)")) -> (read buffer=w1867:string)  [unwired: 1 in, 3 out]
        n1726 = String Subset(string=w1867, offset (0)=0, length (rest)=2 ("length (rest)")) -> (substring=w1866:string)
        n1727 = Match Pattern(string=w1866, regular expression="<>") -> (offset past match=w1863:i32)  [unwired: 1 in, 3 out]
        n1728 = Greater Or Equal?(x=w1863, y=0) -> (x >= y?=w1858:bool)
        n1729 = case shown="True" w1858 {
          tunnel: w1859 -> [_ w1877]
          tunnel: w1868 -> [_ w1876]
          frame False {
          }
          frame True {
            n1730 = VISA Read(VISA resource name=w1877, byte count=u32 32 ("byte count (0)"), error in (no error)=w1876) -> (read buffer=w1875:string)  [unwired: 3 out]
            n1731 = String Subset(string=w1875, offset (0)=0, length (rest)=8 ("length (rest)")) -> (substring=w1879:string)
            n1732 = String Subset(string=w1875, offset (0)=8, length (rest)=8 ("length (rest)")) -> (substring=w1880:string)
            n1733 = Decimal String To Number(string=w1880) -> (number=w1887:i32)  [unwired: 2 in, 1 out]
            n1734 = Decimal String To Number(string=w1879) -> (number=w1883:i32)  [unwired: 2 in, 1 out]
            n1735 = Divide(x=w1887, y=10000) -> ()  [unwired: 1 out]
            n1736 = Divide(x=w1883, y=1000000) -> ()  [unwired: 1 out]
          }
        }
        n1737 = local read "Quit"() -> (w1856:bool)
      }
    }
    frame Enabled {
    }
  }
  n1738 = Tick Count (ms)() -> (millisecond timer value=w6:u32)
  n1739 = while {
    shift-right: [w1933] -> _
    shift-left: w8 -> [w1937]
    shift-right: [w1932] -> _
    shift-left: w7 -> [w1936]
    shift-right: [w1931] -> _
    shift-left: w8 -> [w1935]
    shift-right: [w1930] -> _
    shift-left: w7 -> [w1934]
    shift-right: [w1928] -> _
    shift-left: w6 -> [w1929]
    shift-right: [w1925] -> _
    shift-left: w5 -> [w1926]
    shift-right: [w1924] -> _
    shift-left: w5 -> [w1927]
    shift-right: [w1917] -> _
    shift-left: w5 -> [w1923]
    shift-right: [w1916] -> _
    shift-left: w5 -> [w1922]
    shift-right: [w1915] -> _
    shift-left: w5 -> [w1921]
    shift-right: [w1914] -> _
    shift-left: w5 -> [w1920]
    shift-right: [w1913] -> _
    shift-left: w5 -> [w1919]
    shift-right: [w1912] -> _
    shift-left: w5 -> [w1918]
    shift-right: [w1911] -> _
    shift-left: w5 -> [w1905]
    shift-right: [w1910] -> _
    shift-left: w5 -> [w1904]
    shift-right: [w1909] -> _
    shift-left: w5 -> [w1903]
    shift-right: [w1908] -> _
    shift-left: w5 -> [w1902]
    shift-right: [w1907] -> _
    shift-left: w5 -> [w1901]
    shift-right: [w1906] -> _
    shift-left: w5 -> [w1900]
    shift-right: [w1891] -> _
    shift-left: w5 -> [w1894]
    shift-right: [w1890] -> _
    shift-left: w5 -> [w1893]
    shift-right: [w1889] -> _
    shift-left: w5 -> [w1892]
    stop <- w1939 stop-if-true
    n1740 = local read "Read UNO"() -> (w1898:string)
    n1741 = local read "Error  2"() -> (w1938:errorcluster)
    n1742 = String Length(string=w1898) -> (length=w1897:i32)
    n1743 = call <vilib>:"Trim Whitespace.vi"("string"=w1898) -> ("trimmed string"=w1899:string)  [unwired: 1 in]
    n1744 = Greater Or Equal?(x=w1897, y=23) -> (x >= y?=w1895:bool)
    n1745 = case shown="No Error" w1938 {
      tunnel: w1937 -> [w1985 w2081]
      tunnel: w1936 -> [w1984 w2080]
      tunnel: w1935 -> [w1983 w2079]
      tunnel: w1934 -> [w1982 w2078]
      tunnel: [w1981 w2081] -> w1933
      tunnel: [w1980 w2080] -> w1932
      tunnel: [w1979 w2079] -> w1931
      tunnel: [w1978 w2078] -> w1930
      tunnel: w1929 -> [w1977 w2077]
      tunnel: [w1976 w2077] -> w1928
      tunnel: w1926 -> [w1975 w2076]
      tunnel: w1927 -> [w1974 w2075]
      tunnel: [w1973 w2076] -> w1925
      tunnel: [w1972 w2075] -> w1924
      tunnel: w1923 -> [w1971 w2074]
      tunnel: w1922 -> [w1970 w2073]
      tunnel: w1921 -> [w1969 w2072]
      tunnel: w1920 -> [w1968 w2071]
      tunnel: w1919 -> [w1967 w2070]
      tunnel: w1918 -> [w1966 w2069]
      tunnel: [w1965 w2074] -> w1917
      tunnel: [w1964 w2073] -> w1916
      tunnel: [w1963 w2072] -> w1915
      tunnel: [w1962 w2071] -> w1914
      tunnel: [w1961 w2070] -> w1913
      tunnel: [w1960 w2069] -> w1912
      tunnel: w1905 -> [w1959 w2068]
      tunnel: [w1958 w2068] -> w1911
      tunnel: [w1957 w2064] -> w1910
      tunnel: [w1956 w2063] -> w1909
      tunnel: [w1955 w2067] -> w1908
      tunnel: [w1954 w2066] -> w1907
      tunnel: [w1953 w2065] -> w1906
      tunnel: w1904 -> [w1952 w2067]
      tunnel: w1903 -> [w1951 w2066]
      tunnel: w1902 -> [w1950 w2065]
      tunnel: w1901 -> [w1949 w2064]
      tunnel: w1900 -> [w1948 w2063]
      tunnel: w1899 -> [w1947 _]
      tunnel: w1895 -> [w1946 _]
      tunnel: w1894 -> [w1945 w2062]
      tunnel: w1893 -> [w1944 w2061]
      tunnel: w1892 -> [w1943 w2060]
      tunnel: [w1942 w2062] -> w1891
      tunnel: [w1941 w2061] -> w1890
      tunnel: [w1940 w2060] -> w1889
      frame No Error {
        n1746 = case shown="True" w1946 {
          tunnel: w1985 -> [w2001 w2053]
          tunnel: w1984 -> [w2000 w2052]
          tunnel: w1983 -> [w1999 w2051]
          tunnel: w1982 -> [w1998 w2050]
          tunnel: [w2001 w2049] -> w1981
          tunnel: [w2000 w2048] -> w1980
          tunnel: [w1999 w2047] -> w1979
          tunnel: [w1998 w2046] -> w1978
          tunnel: w1977 -> [w1997 w2044]
          tunnel: [w1997 w2043] -> w1976
          tunnel: w1975 -> [w1996 w2042]
          tunnel: w1974 -> [w1995 w2041]
          tunnel: [w1996 w2040] -> w1973
          tunnel: [w1995 w2039] -> w1972
          tunnel: w1971 -> [w1994 w2038]
          tunnel: w1970 -> [w1993 w2037]
          tunnel: w1969 -> [w1992 w2036]
          tunnel: w1968 -> [w1991 w2035]
          tunnel: w1967 -> [w1990 w2034]
          tunnel: w1966 -> [w1989 w2033]
          tunnel: [w1994 w2032] -> w1965
          tunnel: [w1993 w2031] -> w1964
          tunnel: [w1992 w2030] -> w1963
          tunnel: [w1991 w2029] -> w1962
          tunnel: [w1990 w2028] -> w1961
          tunnel: [w1989 w2027] -> w1960
          tunnel: w1959 -> [w2007 w2026]
          tunnel: [w2007 w2025] -> w1958
          tunnel: [w2004 w2024] -> w1957
          tunnel: [w2003 w2023] -> w1956
          tunnel: [w2006 w2022] -> w1955
          tunnel: [w2002 w2021] -> w1954
          tunnel: [w2005 w2020] -> w1953
          tunnel: w1952 -> [w2006 w2019]
          tunnel: w1951 -> [w2005 w2018]
          tunnel: w1950 -> [w2004 w2017]
          tunnel: w1949 -> [w2003 w2016]
          tunnel: w1948 -> [w2002 w2015]
          tunnel: w1947 -> [_ w2014]
          tunnel: w1945 -> [w1988 w2013]
          tunnel: w1944 -> [w1987 w2012]
          tunnel: w1943 -> [w1986 w2011]
          tunnel: [w1988 w2010] -> w1942
          tunnel: [w1987 w2009] -> w1941
          tunnel: [w1986 w2008] -> w1940
          frame False {
          }
          frame True {
            n1747 = Tick Count (ms)() -> (millisecond timer value=w2045:u32)
            n1748 = String To Byte Array(string=w2014) -> (unsigned byte array=w2058:u8[])
            n1749 = Array Size(array=w2058) -> (size(s)=w2057:i32)
            n1750 = formula code="// --- INTERNAL VARIABLE DECLARATIONS ---\nint i = 0;\nint k = 0;\nint start_idx = -1;\nint end_idx = -1;\nint phase = 0;\nint sign0 = 1;\nint sign1 = 1;\nint ch0_val = 0;   \nint ch1_val = 0;   \nfloat ch0_raw = 0.0;\nfloat ch1_raw = 0.0;\nfloat temp0 = 0.0;\nfloat temp1 = 0.0;\nfloat ch0_clean = 0.0;\nfloat ch1_clean = 0.0;\n\nint valid_samples = 0; // FIX: Track if we actually parsed new data this window\nfloat max_allowed_bits = 8388607.0; // FIX: Change this to match your ADC max value\n\n// Temporal intermediate variables for calculation smoothing\nfloat raw_p2p_v = 0.0;\nfloat raw_friction = 0.0;\nfloat raw_cof = 0.0;\n\n// Temporal intermediate variables for Piezo voltage translations\nfloat piezo_min_v = 0.0;\nfloat piezo_max_v = 0.0;\n\n// Initialize output variables to current shift register states right away\nout_LVDT_Min_V = in_LVDT_Min_V;\nout_LVDT_Max_V = in_LVDT_Max_V;\nout_LVDT_P2P_V = in_LVDT_P2P_V;\nout_Piezo_P2P = in_Piezo_P2P;\nout_Friction_N = in_Friction_N;\nout_COF = in_COF;\nwindow_ready = 0;\n\n// --- STEP 1: PARSE EVERY STRING IN THE BYTE ARRAY ---\nif (array_size > 2) {\n    for (i = 0; i < array_size - 1; i++) {\n        if (raw_bytes[i] == 42) { // '*' character detected\n            start_idx = i;\n        }\n        \n        // Match standard delimiter sequence \";&\" or end window character\n        if (raw_bytes[i] == 59 && raw_bytes[i+1] == 38 && start_idx != -1) { \n            end_idx = i;\n            ch0_val = 0;\n            ch1_val = 0;\n            sign0 = 1;\n            sign1 = 1;\n            phase = 0; \n\n            for (k = start_idx + 1; k < end_idx; k++) {\n                if (raw_bytes[k] == 45) { // '-' sign\n                    if (phase == 0) sign0 = -1;\n                    else sign1 = -1;\n                }\n                else if (raw_bytes[k] == 43) { // '+' sign\n                    if (phase == 0) sign0 = 1;\n                    else sign1 = 1;\n                }\n                else if (raw_bytes[k] == 59) { // ';' delimiter\n                    phase = 1; \n                }\n                else if (raw_bytes[k] >= 48 && raw_bytes[k] <= 57) { // Numeric ASCII digits\n                    if (phase == 0) {\n                        ch0_val = (ch0_val * 10) + (raw_bytes[k] - 48);\n                    } else {\n                        ch1_val = (ch1_val * 10) + (raw_bytes[k] - 48);\n                    }\n                }\n            }\n\n            // Implicit type conversion\n            ch0_raw = ch0_val * sign0 * 1.0;\n            ch1_raw = ch1_val * sign1 * 1.0;\n\n            // FIX: Sanity check / Hard-clamping to catch sudden massive ASCII noise spikes\n            if (ch0_raw > max_allowed_bits)  ch0_raw = max_allowed_bits;\n            if (ch0_raw < -max_allowed_bits) ch0_raw = -max_allowed_bits;\n            if (ch1_raw > max_allowed_bits)  ch1_raw = max_allowed_bits;\n            if (ch1_raw < -max_allowed_bits) ch1_raw = -max_allowed_bits;\n\n            // --- STEP 2: 3-SAMPLE MEDIAN FILTER ---\n            m0_2 = m0_1; m0_1 = m0_0; m0_0 = ch0_raw;\n            float s0_0 = m0_0; float s0_1 = m0_1; float s0_2 = m0_2;\n            if (s0_0 > s0_1) { temp0 = s0_0; s0_0 = s0_1; s0_1 = temp0; }\n            if (s0_1 > s0_2) { temp0 = s0_1; s0_1 = s0_2; s0_2 = temp0; }\n            if (s0_0 > s0_1) { temp0 = s0_0; s0_0 = s0_1; s0_1 = temp0; }\n            ch0_clean = s0_1;\n\n            m1_2 = m1_1; m1_1 = m1_0; m1_0 = ch1_raw;\n            float s1_0 = m1_0; float s1_1 = m1_1; float s1_2 = m1_2;\n            if (s1_0 > s1_1) { temp1 = s1_0; s1_0 = s1_1; s1_1 = temp1; }\n            if (s1_1 > s1_2) { temp1 = s1_1; s1_1 = s1_2; s1_2 = temp1; }\n            if (s1_0 > s1_1) { temp1 = s1_0; s1_0 = s1_1; s1_1 = temp1; }\n            ch1_clean = s1_1;\n\n            // --- STEP 3: EXPONENTIAL FILTER (STREAM LEVEL) ---\n            if (ch0_filt == 0.0) ch0_filt = ch0_clean;\n            if (ch1_filt == 0.0) ch1_filt = ch1_clean;\n\n            ch0_filt = ch0_filt + (ch0_clean - ch0_filt) * 0.125;\n            ch1_filt = ch1_filt + (ch1_clean - ch1_filt) * 0.125;\n\n            // --- STEP 4: MIN/MAX WINDOW CONTINUOUS ACCUMULATION ---\n            if (ch0_filt > max_ch0) max_ch0 = ch0_filt;\n            if (ch0_filt < min_ch0) min_ch0 = ch0_filt;\n            if (ch1_filt > max_ch1) max_ch1 = ch1_filt;\n            if (ch1_filt < min_ch1) min_ch1 = ch1_filt;\n\n            valid_samples++; // FIX: Successfully parsed and accumulated a clean point\n            start_idx = -1; \n        }\n    }\n}\n\n// --- STEP 5: WINDOW EVALUATION ENGINE ---\n// FIX: Condition updated to verify that valid samples exist for both channels\nif (((current_time_ms - start_time_ms) >= 50) && (valid_samples > 0) && (min_ch0 < 9000000.0) && (min_ch1 < 9000000.0)) {\n    window_ready = 1;\n\n    // Linear Bit-to-Voltage Transformations (LVDT - Channel 0)\n    out_LVDT_Min_V = (min_ch0 * VREF) / 8388607.0;\n    out_LVDT_Max_V = (max_ch0 * VREF) / 8388607.0;\n    raw_p2p_v = out_LVDT_Max_V - out_LVDT_Min_V;\n\n    // Linear Bit-to-Voltage Transformations (Piezo - Channel 1)\n    piezo_min_v = (min_ch1 * VREF) / 8388607.0;\n    piezo_max_v = (max_ch1 * VREF) / 8388607.0;\n    \n    // Assign Peak-to-Peak Voltage directly to output indicator (Matches Python logic)\n    out_Piezo_P2P = piezo_max_v - piezo_min_v;\n    \n    // Force scaling calculations using Voltage delta * Newtons/Volt Factor\n    raw_friction = out_Piezo_P2P * PIEZO_CAL_FACTOR ;\n    raw_cof = raw_friction / NORMAL_FORCE;\n\n    // --- STEP 6: OUTPUT METRIC SMOOTHING (Low-Pass Filter Alpha = 0.05) ---\n    // Seed initial historical metrics if first loop iteration\n    if (hist_LVDT_P2P == 0.0) hist_LVDT_P2P = raw_p2p_v;\n    if (hist_Friction == 0.0) hist_Friction = raw_friction;\n    if (hist_COF == 0.0)      hist_COF = raw_cof;\n\n    // Apply exponential output dampening\n    hist_LVDT_P2P = hist_LVDT_P2P + (raw_p2p_v - hist_LVDT_P2P) * 0.05;\n    hist_Friction = hist_Friction + (raw_friction - hist_Friction) * 0.05; // Note: Can drop to 0.02 for more aggressive damping\n    hist_COF      = hist_COF + (raw_cof - hist_COF) * 0.05;\n\n    // Direct smoothed parameters out to UI Indicators\n    out_LVDT_P2P_V = hist_LVDT_P2P;\n    out_Friction_N = hist_Friction;\n    out_COF        = hist_COF;\n\n    // Reset tracking targets to extreme boundaries safely\n    min_ch0 = 9999999.0;\n    max_ch0 = -9999999.0;\n    min_ch1 = 9999999.0;\n    max_ch1 = -9999999.0;\n\n    valid_samples = 0; // FIX: Reset counter for next time frame\n    start_time_ms = current_time_ms;\n}"("raw_bytes"=w2058, "array_size"=w2057, "VREF"="VREF", "PIEZO_CAL_FACTOR"="PIEZO_CAL_FACTOR", "NORMAL_FORCE"="NORMAL_FORCE", "min_ch0"=w2053, "max_ch0"=w2052, "min_ch1"=w2051, "max_ch1"=w2050, "current_time_ms"=w2045, "start_time_ms"=w2044, "ch0_filt"=w2042, "ch1_filt"=w2041, "m0_0"=w2038, "m0_1"=w2037, "m0_2"=w2036, "m1_0"=w2035, "m1_1"=w2034, "m1_2"=w2033, "in_LVDT_Min_V"=w2026, "in_LVDT_Max_V"=w2019, "in_LVDT_P2P_V"=w2018, "in_Piezo_P2P"=w2017, "in_Friction_N"=w2016, "in_COF"=w2015, "hist_LVDT_P2P"=w2013, "hist_Friction"=w2012, "hist_COF"=w2011) -> ("window_ready"=→"Valid_data":dbl, "out_LVDT_Min_V"=w2025:dbl, "out_LVDT_Max_V"=w2024:dbl, "out_LVDT_P2P_V"=w2023:dbl, "out_Piezo_P2P"=w2022:dbl, "out_Friction_N"=w2021:dbl, "out_COF"=w2020:dbl, "min_ch0"=w2049:dbl, "max_ch0"=w2048:dbl, "min_ch1"=w2047:dbl, "max_ch1"=w2046:dbl, "start_time_ms"=w2043:u32, "ch0_filt"=w2040:dbl, "ch1_filt"=w2039:dbl, "m0_0"=w2032:dbl, "m0_1"=w2031:dbl, "m0_2"=w2030:dbl, "m1_0"=w2029:dbl, "m1_1"=w2028:dbl, "m1_2"=w2027:dbl, "hist_LVDT_P2P"=w2010:dbl, "hist_Friction"=w2009:dbl, "hist_COF"=w2008:dbl)
            "LVDT MIN" <- w2025
            "LVDT MAX" <- w2024
            "LVDT Peak" <- w2023
            "pizo raw" <- w2022
            "cof" <- w2020
            "Frictioin Force Raw" <- w2021
          }
        }
      }
      frame Error {
      }
    }
    n1751 = local read "Quit"() -> (w1939:bool)
  }
  n1752 = disable-structure shown="Disabled" {
    disable-tunnel: errorcluster {"status"=TRUE, "code"=0, "source"="Init"} ("error IO") -> [w2084 _]
    disable-tunnel: [w2082 _] -> w47
    frame Disabled {
      n1753 = while {
        shift-right: [w2100] -> w2086
        shift-left: _ -> [w2091]
        shift-right: [w2099] -> w2085
        shift-left: w2084 -> [w2093]
        tunnel: [w2088] -> w2082
        tunnel: [w2098] -> _
        i -> [w2098]
        stop <- w2088 stop-if-true
        n1754 = local read "Port 1a"() -> (w2094:bool)
        n1755 = local read "Port 3"() -> (w2095:bool)
        n1756 = local read "Com Port 1"() -> (w2092:refnum<visa-resource-name>)
        n1757 = Or(x=w2095, y=w2094) -> (x .or. y?=w2097:bool)
        n1758 = Unbundle(w2093) -> ("status"=→"Port 3":bool)  [unwired: 2 out]